vi "TLB Native Dynamic Events ver 0.26d.vi"() -> ()   [LabVIEW 2018] (continued)
      tunnel: [_ _ _ _ _ _ _ _ _ _ _ _ _ _ _ _ _ _ _ _ _ _ _ _ _ _ _ _ _ _ _ _ _ _ _ w3525 w3555 _ _ _ _ _ _ _ _ _ _ _ _ _ _ _ _ _ _ _ _] -> w221
      tunnel: w219 -> [w2959 w2972 w2984 w2999 w3018 w3033 w3048 w3062 w3076 w3092 w3107 w3121 w3132 w3149 w3167 w3185 w3201 w3220 w3232 w3262 w3275 w3288 w3303 w3314 w3333 w3353 w3388 w3419 w3432 w3445 w3456 w3468 w3484 w3500 w3512 w3524 w3559 w3570 w3582 w3603 w3614 w3625 w3638 w3651 w3664 w3677 w3690 w3705 w3721 w3734 w3750 w3766 w3782 w3799 w3812 w3832 w3852]
      tunnel: [w2959 w2972 w2984 w2999 w3018 w3033 w3048 w3062 w3076 w3092 w3107 w3121 w3132 w3149 w3167 w3185 w3201 w3220 w3232 w3262 w3275 w3288 w3303 w3314 w3333 w3353 w3388 w3419 w3432 w3445 w3456 w3468 w3484 w3500 w3512 w3524 w3559 w3570 w3582 w3603 w3614 w3625 w3638 w3651 w3664 w3677 w3690 w3705 w3721 w3734 w3750 w3766 w3782 w3799 w3812 w3832 w3852] -> w218
      tunnel: w214 -> [w2958 w2971 w2983 w2998 w3017 w3032 w3047 w3061 w3075 w3091 w3106 w3120 w3131 w3148 w3166 w3182 w3200 w3219 w3231 w3261 w3274 w3287 w3302 w3313 w3328 w3346 w3381 w3418 w3431 w3444 w3455 w3467 w3483 w3499 w3511 w3523 w3553 w3569 w3581 w3602 w3613 w3624 w3637 w3650 w3663 w3676 w3689 w3704 w3720 w3733 w3749 w3765 w3781 w3798 w3811 w3831 w3846]
      tunnel: [w2958 w2971 w2983 w2998 w3017 w3032 w3047 w3061 w3075 w3091 w3106 w3120 w3131 w3148 w3166 w3182 w3200 w3219 w3231 w3261 w3274 w3287 w3302 w3313 w3327 w3346 w3381 w3418 w3431 w3444 w3455 w3467 w3483 w3499 w3511 w3523 w3546 w3569 w3581 w3601 w3613 w3624 w3637 w3650 w3663 w3676 w3689 w3704 w3720 w3733 w3749 w3765 w3781 w3798 w3811 w3831 w3845] -> w213
      frame "Exit" {
        # ">>State Logic  >>"
        # ">>> Time cluster >>>"
        # ">>> Yaw >>>"
        # ">>> Stepper position >>>"
        # ">>> Encoders >>>"
        # ">>> Object detection >>>"
        # ">>> Ultrasonic Sensors Detect >>>"
        n70 = call "Imaq Dispose"("All Images? (No)"=TRUE) -> ()  [unwired: 5 in, 1 out]
      }
      frame "----Movement States----" {
        # ">>State Logic  >>"
        # ">>> Time cluster >>>"
        # ">>> Yaw >>>"
        # ">>> Stepper position >>>"
        # ">>> Encoders >>>"
        # ">>> Object detection >>>"
        # ">>> Ultrasonic Sensors Detect >>>"
      }
      frame "FORWARD" {
        # ">>State Logic  >>"
        # ">>> Time cluster >>>"
        # ">>> Yaw >>>"
        # ">>> Stepper position >>>"
        # ">>> Encoders >>>"
        # ">>> Object detection >>>"
        # ">>> Ultrasonic Sensors Detect >>>"
        n71 = Unbundle By Name(w2991) -> ("Yaw"=w2987:dbl)
        n72 = call "MOTOR CONTROL WITH PID AE.vi"("Yaw"=w2987, "Speed"=50.0, "Direction"=MOTOR_CONTROL_WITH_PID_AE_DIRECTION_TYPE_DEF."y-axis movement", "AE Mode"=MOTOR_CONTROL_WITH_PID_AE_DATA_MODE_TYPE_DEF."Write to AE") -> ()  [unwired: 1 out]
      }
      frame "FORWARD - IR ASSIST" {
        # "Algorithm sensitivity"
        # "Distance to maintain from wall"
        # ">>State Logic  >>"
        # ">>> Time cluster >>>"
        # ">>> Yaw >>>"
        # ">>> Stepper position >>>"
        # ">>> Encoders >>>"
        # ">>> Object detection >>>"
        # ">>> Ultrasonic Sensors Detect >>>"
        n73 = Unbundle By Name(w3006) -> ("Left IR Sensor"=w3005:dbl)
        n74 = Subtract(x=w3005, y=10.0) -> (x-y=w3003:dbl)
        n75 = Multiply(x=w3003, y=0.2) -> (x*y=w3001:dbl)
        n76 = call "MOTOR CONTROL WITH PID AE.vi"("Yaw"=w3001, "Speed"=35.0, "Direction"=MOTOR_CONTROL_WITH_PID_AE_DIRECTION_TYPE_DEF."y-axis movement", "AE Mode"=MOTOR_CONTROL_WITH_PID_AE_DATA_MODE_TYPE_DEF."Write to AE") -> ()  [unwired: 1 out]
      }
      frame "LEFT" {
        # ">>State Logic  >>"
        # ">>> Time cluster >>>"
        # ">>> Yaw >>>"
        # ">>> Stepper position >>>"
        # ">>> Encoders >>>"
        # ">>> Object detection >>>"
        # ">>> Ultrasonic Sensors Detect >>>"
        n77 = Unbundle By Name(w3025) -> ("Yaw"=w3022:dbl)
        n78 = call "MOTOR CONTROL WITH PID AE.vi"("Yaw"=w3022, "Speed"=-20.0, "Direction"=MOTOR_CONTROL_WITH_PID_AE_DIRECTION_TYPE_DEF."x-axis movement", "AE Mode"=MOTOR_CONTROL_WITH_PID_AE_DATA_MODE_TYPE_DEF."Write to AE") -> ()  [unwired: 1 out]
      }
      frame "RIGHT" {
        # ">>> Time cluster >>>"
        # ">>> Yaw >>>"
        # ">>> Stepper position >>>"
        # ">>> Encoders >>>"
        # ">>> Object detection >>>"
        # ">>> Ultrasonic Sensors Detect >>>"
        n79 = Unbundle By Name(w3040) -> ("Yaw"=w3036:dbl)
        n80 = call "MOTOR CONTROL WITH PID AE.vi"("Yaw"=w3036, "Speed"=20.0, "Direction"=MOTOR_CONTROL_WITH_PID_AE_DIRECTION_TYPE_DEF."x-axis movement", "AE Mode"=MOTOR_CONTROL_WITH_PID_AE_DATA_MODE_TYPE_DEF."Write to AE") -> ()  [unwired: 1 out]
      }
      frame "R-ACW" {
        # ">>> IR Sensors >>>"
        # ">>> Time cluster >>>"
        # ">>> Yaw >>>"
        # ">>> Stepper position >>>"
        # ">>> Encoders >>>"
        # ">>> Object detection >>>"
        # ">>> Ultrasonic Sensors Detect >>>"
        n81 = call "MOTOR CONTROL WITH PID AE.vi"("Speed"=10.0, "Direction"=MOTOR_CONTROL_WITH_PID_AE_DIRECTION_TYPE_DEF."rotation", "AE Mode"=MOTOR_CONTROL_WITH_PID_AE_DATA_MODE_TYPE_DEF."Write to AE") -> ()  [unwired: 1 in, 1 out]
      }
      frame "R-CW" {
        (unwired) -0.2 ("Speed")
        # ">>> Time cluster >>>"
        # ">>> Yaw >>>"
        # ">>> Stepper position >>>"
        # ">>> Encoders >>>"
        # ">>> Object detection >>>"
        # ">>> Ultrasonic Sensors Detect >>>"
        n82 = call "MOTOR CONTROL WITH PID AE.vi"("Speed"=-10.0, "Direction"=MOTOR_CONTROL_WITH_PID_AE_DIRECTION_TYPE_DEF."rotation", "AE Mode"=MOTOR_CONTROL_WITH_PID_AE_DATA_MODE_TYPE_DEF."Write to AE") -> ()  [unwired: 1 in, 1 out]
      }
      frame "X AXIS - SLOW" {
        # ">>> Line Sensor Cluster>>>"
        # ">>> IR Sensors >>>"
        # ">>> Time cluster >>>"
        # ">>> Yaw >>>"
        # ">>> Stepper position >>>"
        # ">>> Encoders >>>"
        # ">>> Object detection >>>"
        # ">>> Ultrasonic Sensors Detect >>>"
        n83 = Unbundle By Name(w3079) -> ("xSpeed"=w3078:dbl)
        n84 = Unbundle By Name(w3084) -> ("Yaw"=w3081:dbl)
        n85 = call "MOTOR CONTROL WITH PID AE.vi"("Yaw"=w3081, "Speed"=w3078, "Direction"=MOTOR_CONTROL_WITH_PID_AE_DIRECTION_TYPE_DEF."x-axis movement", "AE Mode"=MOTOR_CONTROL_WITH_PID_AE_DATA_MODE_TYPE_DEF."Write to AE") -> ()  [unwired: 1 out]
      }
      frame "REVERSE" {
        # ">>> Time cluster >>>"
        # ">>> Yaw >>>"
        # ">>> Stepper position >>>"
        # ">>> Encoders >>>"
        # ">>> Object detection >>>"
        # ">>> Ultrasonic Sensors Detect >>>"
        n86 = Unbundle By Name(w3099) -> ("Yaw"=w3095:dbl)
        n87 = call "MOTOR CONTROL WITH PID AE.vi"("Yaw"=w3095, "Speed"=-50.0, "Direction"=MOTOR_CONTROL_WITH_PID_AE_DIRECTION_TYPE_DEF."y-axis movement", "AE Mode"=MOTOR_CONTROL_WITH_PID_AE_DATA_MODE_TYPE_DEF."Write to AE") -> ()  [unwired: 1 out]
      }
      frame "STOP" {
        n88 = Wait (ms)(milliseconds to wait=u32 100) -> ()  [unwired: 1 out]
        n89 = call "MOTOR CONTROL WITH PID AE.vi"("Direction"=MOTOR_CONTROL_WITH_PID_AE_DIRECTION_TYPE_DEF."stop", "AE Mode"=MOTOR_CONTROL_WITH_PID_AE_DATA_MODE_TYPE_DEF."Write to AE") -> ()  [unwired: 2 in, 1 out]
      }
      frame "----SENSOR READING---- " {
      }
      frame "READ ENCODERS" {
        # ">>> Time cluster >>>"
        # ">>> Yaw >>>"
        # ">>> Stepper position >>>"
        # ">>> Object detection >>>"
        # ">>> Current encoder distance >>>"
        # ">>> Ultrasonic Sensors Detect >>>"
        n90 = call "MOTOR CONTROL WITH PID AE.vi"("AE Mode"=MOTOR_CONTROL_WITH_PID_AE_DATA_MODE_TYPE_DEF."Read from AE") -> ("Speed & distance"=w3138:T15)  [unwired: 3 in]
        n91 = Unbundle By Name(w3138) -> ("xDistance"=w3137:dbl, "yDistance"=w3136:dbl, "wDistance"=w3135:dbl)
        n92 = Bundle By Name(cluster=w3145, "xDistance"=w3137, "yDistance"=w3136, "wDistance"=w3135) -> (w3144:T8)
      }
      frame "READ ULTRASONIC" {
        (unwired) navX_type_def."Read Values" ("Mode")
        (unwired) MOTOR_CONTROL_NO_PID_Type_Def."Latch" ("Direction")
        # ">>> Line Sensor Cluster>>>"
        # ">>> IR Sensors >>>"
        # ">>State Logic  >>"
        # ">>> Time cluster >>>"
        # ">>> Ultrasonic Sensors Detect >>>"
        # ">>> Object detection >>>"
        # ">>> Encoders >>>"
        # ">>> Stepper position >>>"
        # ">>> Yaw >>>"
        n93 = call "Arduino Interfacing VI.vi"("AE Mode"=Arduino_Interfacing."Read From Arduino") -> ("Arduino Data"=w3158:T17)  [unwired: 3 in, 1 out]
        n94 = Unbundle By Name(w3158) -> ("PING A"=w3157:u8, "PING B"=w3156:u8, "PING C"=w3155:u8, "PING D"=w3154:u8)
        n95 = Bundle By Name(cluster=w3164, "PING_A"=w3157, "PING_B"=w3156, "PING_C"=w3155, "PING_D"=w3154) -> (w3165:T9)
      }
      frame "READ NAVX" {
        # ">> Item Selection Bias >>"
        # ">>State Logic  >>"
        # ">>> Line Sensor Cluster>>>"
        # ">>> IR Sensors >>>"
        # ">>> Time cluster >>>"
        # ">>> Yaw >>>"
        # ">>> Ultrasonic Sensors Detect >>>"
        # ">>> Object detection >>>"
        # ">>> Encoders >>>"
        # ">>> Stepper position >>>"
        n96 = call "navX reading VI.vi"("Mode"=navX_type_def."Read Values") -> ("NavX Readings"=w3171:T16)  [unwired: 2 in, 3 out]
        n97 = Unbundle By Name(w3171) -> ("Heading"=w3170:dbl)
        n98 = Unbundle By Name(w3171) -> ("Yaw"=w3174:dbl)
        n99 = Bundle By Name(cluster=w3176, "Yaw"=w3174, "Compass"=w3170) -> (w3175:T6)
      }
      frame "READ IR" {
        w3184 = T41 [enum."B/AI2"] items=["Not Connected", "AudioIn/Left", "AudioIn/Right", "C/AI0", "C/AI1", "A/AI0", "A/AI1", "A/AI2", "A/AI3", "A/AI4", "A/AI5", "A/AI6", "A/AI7", "B/AI0", "B/AI1", "B/AI2", "B/AI3", "B/AI4", "B/AI5", "B/AI6", "B/AI7", "AI/AI0", "AI/AI1", "AI/AI2", "AI/AI3", "A/AI0 (DIFF)", "A/AI1 (DIFF)", "A/AI2 (DIFF)", "A/AI3 (DIFF)", "B/AI0 (DIFF)", "B/AI1 (DIFF)", "B/AI2 (DIFF)", "B/AI3 (DIFF)"] ("AI Channel")
        w3188 = T41 [enum."B/AI1"] items=["Not Connected", "AudioIn/Left", "AudioIn/Right", "C/AI0", "C/AI1", "A/AI0", "A/AI1", "A/AI2", "A/AI3", "A/AI4", "A/AI5", "A/AI6", "A/AI7", "B/AI0", "B/AI1", "B/AI2", "B/AI3", "B/AI4", "B/AI5", "B/AI6", "B/AI7", "AI/AI0", "AI/AI1", "AI/AI2", "AI/AI3", "A/AI0 (DIFF)", "A/AI1 (DIFF)", "A/AI2 (DIFF)", "A/AI3 (DIFF)", "B/AI0 (DIFF)", "B/AI1 (DIFF)", "B/AI2 (DIFF)", "B/AI3 (DIFF)"] ("AI Channel")
        w3193 = T41 [enum."B/AI0"] items=["Not Connected", "AudioIn/Left", "AudioIn/Right", "C/AI0", "C/AI1", "A/AI0", "A/AI1", "A/AI2", "A/AI3", "A/AI4", "A/AI5", "A/AI6", "A/AI7", "B/AI0", "B/AI1", "B/AI2", "B/AI3", "B/AI4", "B/AI5", "B/AI6", "B/AI7", "AI/AI0", "AI/AI1", "AI/AI2", "AI/AI3", "A/AI0 (DIFF)", "A/AI1 (DIFF)", "A/AI2 (DIFF)", "A/AI3 (DIFF)", "B/AI0 (DIFF)", "B/AI1 (DIFF)", "B/AI2 (DIFF)", "B/AI3 (DIFF)"] ("AI Channel")
        # ">>> Line Sensor Cluster>>>"
        # ">>> IR Sensors >>>"
        # ">>State Logic  >>"
        # ">>> Time cluster >>>"
        # ">>> Ultrasonic Sensors Detect >>>"
        # ">>> Object detection >>>"
        # ">>> Encoders >>>"
        # ">>> Stepper position >>>"
        # ">>> Yaw >>>"
        n100 = call <vilib>:"Sharp IR.vi"("AI Channel"=w3193) -> ("Sharp IR Distance"=w3189:dbl)  [unwired: 8 in, 2 out]
        n101 = call <vilib>:"Sharp IR.vi"("AI Channel"=w3188) -> ("Sharp IR Distance"=w3187:dbl)  [unwired: 8 in, 2 out]
        n102 = call <vilib>:"Sharp IR.vi"("AI Channel"=w3184) -> ("Sharp IR Distance"=w3183:dbl)  [unwired: 8 in, 2 out]
        n103 = Bundle By Name(cluster=w3191, "Left IR Sensor"=w3189, "Arm IR Sensor"=w3187, "Bottom IR Sensor"=w3183) -> (w3190:T5)
      }
      frame "READ LINE SENSOR" {
        # ">>> IR Sensors >>>"
        # ">>> Line Sensor Cluster>>>"
        # ">>State Logic  >>"
        # ">>> Time cluster >>>"
        # ">>> Object detection >>>"
        # ">>> Yaw >>>"
        # ">>> Ultrasonic Sensors Detect >>>"
        # ">>> Encoders >>>"
        # ">>> Stepper position >>>"
        n104 = call "Line Sensor AE.vi"("AE State"=Line_Sensor_AE_Type_Def."READ FROM LINE SENSORS") -> ("Line Detected?"=w3207:bool, "Line Sensor Raw Values"=w3206:T43)
        n105 = Unbundle By Name(w3206) -> ("S1"=w3205:dbl, "S2"=w3204:dbl, "S3"=w3203:dbl, "S4"=w3202:dbl)
        n106 = Bundle By Name(cluster=w3210, "Line Detected?"=w3207, "S1"=w3205, "S2"=w3204, "S3"=w3203, "S4"=w3202) -> (w3209:T4)
      }
      frame "----SYSTEM MODES----" {
        (unwired) I2C_MASTER_Type_Def."Last State" ("Arduino Mode")
        # ">>> Object detection >>>"
        # ">>> Yaw >>>"
        # ">>> Ultrasonic Sensors Detect >>>"
        # ">>> Encoders >>>"
        # ">>> Stepper position >>>"
      }
      frame "INIT" {
        w3254 = u8 0
        w3255 = 0.0
        # ">>> IR Sensors >>>"
        # ">>> IR Sensors >>>"
        # ">>> Line Sensor Cluster>>>"
        # ">>> Time cluster >>>"
        # ">>> Object detection >>>"
        # ">>> Yaw >>>"
        # ">>> Ultrasonic Sensors Detect >>>"
        # ">>> Encoders >>>"
        # ">>> Stepper position >>>"
        # ">>State Logic  >>"
        n107 = call "Arduino Interfacing VI.vi"("AE Mode"=Arduino_Interfacing."Initialize") -> ()  [unwired: 3 in, 2 out]
        n108 = call "FGV Stop.vi"("Init/Read/Write State"=States_for_Action_Engine."Initialize") -> ()  [unwired: 2 in, 2 out]
        n109 = call "Elasped Timer.vi"("Action"=Elapsed_timer_control."Initialize") -> ()  [unwired: 7 in, 4 out]
        n110 = call "MOTOR CONTROL WITH PID AE.vi"("AE Mode"=MOTOR_CONTROL_WITH_PID_AE_DATA_MODE_TYPE_DEF."Init AE") -> ()  [unwired: 3 in, 1 out]
        n111 = call "IMAQ Reference AE.vi"("IMAQ AE States"=IMAQ_Reference_AE."Initialize AE") -> ()  [unwired: 1 in, 2 out]
        n112 = call "Line Sensor AE.vi"("AE State"=Line_Sensor_AE_Type_Def."INIT AE") -> ()  [unwired: 2 out]
        n113 = Bundle By Name(cluster=w3248, "Recognized Object"=FALSE, "Object X coordinate"=0.0, "Object Y coordinate"=0.0) -> (w3247:T11)
        n114 = Bundle By Name(cluster=w3253, "y Stepper Position"=u8 0, "z Stepper Position"=u8 0) -> (w3252:T7)
        n115 = Bundle By Name(cluster=w3257, "xDistance"=w3255, "yDistance"=w3255, "wDistance"=w3255) -> (w3256:T8)
        n116 = Bundle By Name(cluster=w3259, "PING_A"=w3254, "PING_B"=w3254, "PING_C"=w3254, "PING_D"=w3254) -> (w3260:T9)
        n117 = Bundle By Name(cluster=w3243, "Yaw"=0.0) -> (w3242:T6)
        n118 = call "Task 9 basic VI.vi"("AE State"=Task_9_Sates."Initialize") -> ()  [unwired: 1 in, 3 out]
      }
      frame "ARDUINO - ULTRASONIC" {
        # ">>> Time cluster >>>"
        # ">>> Line Sensor Cluster>>>"
        # ">>> Object detection >>>"
        # ">>> Yaw >>>"
        # ">>> Ultrasonic Sensors Detect >>>"
        # ">>> Encoders >>>"
        # ">>> Stepper position >>>"
        # ">>State Logic  >>"
        n119 = call "Arduino Interfacing VI.vi"("Data to Write"=I2C_MASTER_WRITE_NEW_Type_Def."Ultrasonic sensors", "AE Mode"=Arduino_Interfacing."Write to Arduino") -> ()  [unwired: 2 in, 2 out]
      }
      frame "NAVX CALIBRATE" {
        # ">>> Object detection >>>"
        # ">>> Yaw >>>"
        # ">>> Ultrasonic Sensors Detect >>>"
        # ">>> Encoders >>>"
        # ">>> Stepper position >>>"
        # ">>State Logic  >>"
        # "Adds a 15 second delay to the startup process \nfor the NavX to calibrate"
        n120 = Wait (ms)(milliseconds to wait=u32 1000) -> ()  [unwired: 1 out]
      }
      frame "NO ACTION", Default {
        (unwired) u8 0 ("y Stepper value")
        (unwired) TRUE ("Latch")
        (unwired) navX_type_def."Read Values" ("Mode")
        (unwired) MOTOR_CONTROL_NO_PID_Type_Def."Latch" ("Direction")
        # ">>> Object detection >>>"
        # ">>> Yaw >>>"
        # ">>> Ultrasonic Sensors Detect >>>"
        # ">>> Encoders >>>"
        # ">>> Stepper position >>>"
        # ">>State Logic  >>"
        n121 = case shown="4" w3296 {
          tunnel: [0 100] -> w3298
          frame 1, Default {
          }
          frame 4 {
          }
        }
      }
      frame "----RESET CASES----" {
        (unwired) I2C_MASTER_Type_Def."Last State" ("Arduino Mode")
        # ">>> Object detection >>>"
        # ">>> Yaw >>>"
        # ">>> Ultrasonic Sensors Detect >>>"
        # ">>> Encoders >>>"
        # ">>> Stepper position >>>"
        # ">>State Logic  >>"
      }
      frame "RESET ENCODERS" {
        # ">>> Object detection >>>"
        # ">>> Yaw >>>"
        # ">>> Ultrasonic Sensors Detect >>>"
        # ">>> Encoders >>>"
        # ">>> Stepper position >>>"
        # ">>State Logic  >>"
        n122 = call "MOTOR CONTROL WITH PID AE.vi"("Direction"=MOTOR_CONTROL_WITH_PID_AE_DIRECTION_TYPE_DEF."reset encoders", "AE Mode"=MOTOR_CONTROL_WITH_PID_AE_DATA_MODE_TYPE_DEF."Write to AE") -> ()  [unwired: 2 in, 1 out]
      }
      frame "RESET FLAGS" {
        w3326 = FALSE ("Line Detected?")
        # ">>> Line Sensor Cluster>>>"
        # ">>> IR Sensors >>>"
        # ">>> Time cluster >>>"
        # ">>> Object detection >>>"
        # ">>> Yaw >>>"
        # ">>> Ultrasonic Sensors Detect >>>"
        # ">>> Encoders >>>"
        # ">>> Stepper position >>>"
        # ">>> Line Sensor Cluster>>>"
        # ">>> IR Sensors >>>"
        # ">>> Time cluster >>>"
        # ">>> Object detection >>>"
        # ">>> Yaw >>>"
        # ">>> Ultrasonic Sensors Detect >>>"
        # ">>> Encoders >>>"
        # ">>> Stepper position >>>"
        # "Resets BOOLEAN FLAGS only"
        n123 = Wait (ms)(milliseconds to wait=u32 20) -> ()  [unwired: 1 out]
        n124 = Bundle By Name(cluster=w3342, "Recognized Object"=FALSE) -> (w3341:T11)
        n125 = Bundle By Name(cluster=w3332, "Line Detected?"=FALSE) -> (w3331:T4)
        n126 = Bundle By Name(cluster=w3336, "Time up flag"=FALSE) -> (w3335:T3)
        n127 = Bundle By Name(cluster=w3328, "Red"=w3326, "Black"=w3326, "Blue"=w3326, "Yellow"=w3326, "Green"=w3326, "Unknown"=w3326, "Image processing done"=w3326) -> (w3327:T1)
      }
      frame "RESET SENSOR VALUES" {
        w3347 = 0.0 ("S4")
        w3348 = 0.0 ("S4")
        # "Resets SENSOR VALUES only"
        # ">>> Line Sensor Cluster>>>"
        # ">>> IR Sensors >>>"
        # ">>> Time cluster >>>"
        # ">>> Object detection >>>"
        # ">>> Yaw >>>"
        # ">>> Ultrasonic Sensors Detect >>>"
        # ">>> Encoders >>>"
        # ">>> Stepper position >>>"
        # ">>> Line Sensor Cluster>>>"
        # ">>> IR Sensors >>>"
        # ">>> Time cluster >>>"
        # ">>> Object detection >>>"
        # ">>> Yaw >>>"
        # ">>> Ultrasonic Sensors Detect >>>"
        # ">>> Encoders >>>"
        # ">>> Stepper position >>>"
        # "Resets any software variables\nand/or non-critical states"
        n128 = Wait (ms)(milliseconds to wait=u32 20) -> ()  [unwired: 1 out]
        n129 = Bundle By Name(cluster=w3356, "SET TIME TO CHECK"=0.0) -> (w3355:T3)
        n130 = Bundle By Name(cluster=w3372, "Object X coordinate"=0.0, "Object Y coordinate"=0.0) -> (w3371:T11)
        n131 = Bundle By Name(cluster=w3363, "y Stepper Position"=u8 0, "z Stepper Position"=u8 0) -> (w3362:T7)
        n132 = Bundle By Name(cluster=w3350, "Left IR Sensor"=w3347, "Arm IR Sensor"=w3347) -> (w3349:T5)
        n133 = Bundle By Name(cluster=w3368, "xDistance"=0.0, "yDistance"=0.0, "wDistance"=0.0) -> (w3367:T8)
        n134 = Bundle By Name(cluster=w3379, "PING_A"=u8 0, "PING_B"=u8 0, "PING_C"=u8 0, "PING_D"=u8 0) -> (w3378:T9)
        n135 = Bundle By Name(cluster=w3359, "Yaw"=0.0) -> (w3358:T6)
        n136 = Bundle By Name(cluster=w3352, "S1"=w3348, "S2"=w3348, "S3"=w3348, "S4"=w3348) -> (w3351:T4)
      }
      frame "RESET ALL SENSORS" {
        w3382 = 0.0 ("SET TIME TO CHECK")
        # ">>> Line Sensor Cluster>>>"
        # ">>> IR Sensors >>>"
        # ">>> Time cluster >>>"
        # ">>> Object detection >>>"
        # ">>> Yaw >>>"
        # ">>> Ultrasonic Sensors Detect >>>"
        # ">>> Encoders >>>"
        # ">>> Stepper position >>>"
        # ">>> Line Sensor Cluster>>>"
        # ">>> IR Sensors >>>"
        # ">>> Time cluster >>>"
        # ">>> Object detection >>>"
        # ">>> Yaw >>>"
        # ">>> Ultrasonic Sensors Detect >>>"
        # ">>> Encoders >>>"
        # ">>> Stepper position >>>"
        # "Resets ALL SENSOR PARAMTERS"
        n137 = Wait (ms)(milliseconds to wait=u32 20) -> ()  [unwired: 1 out]
        n138 = Bundle By Name(cluster=w3392, "Time up flag"=FALSE, "SET TIME TO CHECK"=0.0) -> (w3391:T3)
        n139 = Bundle By Name(cluster=w3409, "Recognized Object"=FALSE, "Object X coordinate"=0.0, "Object Y coordinate"=0.0) -> (w3408:T11)
        n140 = Bundle By Name(cluster=w3399, "y Stepper Position"=u8 0, "z Stepper Position"=u8 0) -> (w3398:T7)
        n141 = Bundle By Name(cluster=w3387, "Line Detected?"=FALSE) -> (w3386:T4)
        n142 = Bundle By Name(cluster=w3384, "Left IR Sensor"=w3382, "Arm IR Sensor"=w3382) -> (w3383:T5)
        n143 = Bundle By Name(cluster=w3404, "xDistance"=0.0, "yDistance"=0.0, "wDistance"=0.0) -> (w3403:T8)
        n144 = Bundle By Name(cluster=w3416, "PING_A"=u8 0, "PING_B"=u8 0, "PING_C"=u8 0, "PING_D"=u8 0) -> (w3415:T9)
        n145 = Bundle By Name(cluster=w3395, "Yaw"=0.0) -> (w3394:T6)
      }
      frame "RESET YAW" {
        n146 = Wait (ms)(milliseconds to wait=u32 100) -> ()  [unwired: 1 out]
        n147 = call "navX reading VI.vi"("Mode"=navX_type_def."Zero Yaw") -> ()  [unwired: 2 in, 4 out]
      }
      frame "RESET ARM" {
        n148 = call "Arduino Interfacing VI.vi"("Data to Write"=I2C_MASTER_WRITE_NEW_Type_Def."Soft Reset", "AE Mode"=Arduino_Interfacing."Write to Arduino") -> ()  [unwired: 2 in, 2 out]
      }
      frame "--------CAM STATES-------" {
      }
      frame "OPEN IMAQ REF" {
        # ">>> Line Sensor Cluster>>>"
        # ">>State Logic  >>"
        # ">>> Time cluster >>>"
        # ">>> Object detection >>>"
        # ">>> Yaw >>>"
        # ">>> Ultrasonic Sensors Detect >>>"
        # ">>> Encoders >>>"
        # ">>> Stepper position >>>"
        # ">>> IR Sensors >>>"
        n149 = call "IMAQ Reference AE.vi"("IMAQ AE States"=IMAQ_Reference_AE."Initialize AE") -> ()  [unwired: 1 in, 2 out]
      }
      frame "OPEN LOG CAM" {
        n150 = call "Webcam AE.vi"("Session In"=T39 "cam0", "Camera states"=Webcam_AE."Initialize Camera") -> ("error out"=w3473:errorcluster, "Session Out"=w3472:T39)  [unwired: 1 in, 1 out]
        n151 = call "Webcam AE.vi"("error in (no error)"=w3473, "Session In"=w3472, "Camera states"=Webcam_AE."Open Camera") -> ()  [unwired: 3 out]
      }
      frame "OPEN LIFE CAM" {
        n152 = call "Webcam AE.vi"("Session In"=T39 "cam1", "Camera states"=Webcam_AE."Initialize Camera") -> ("error out"=w3489:errorcluster, "Session Out"=w3488:T39)  [unwired: 1 in, 1 out]
        n153 = call "Webcam AE.vi"("error in (no error)"=w3489, "Session In"=w3488, "Camera states"=Webcam_AE."Open Camera") -> ()  [unwired: 3 out]
      }
      frame "CAM ACQ" {
        # ">>State Logic  >>"
        # ">>> Time cluster >>>"
        # ">>> Yaw >>>"
        # ">>> Stepper position >>>"
        # ">>> Encoders >>>"
        # ">>> Object detection >>>"
        # ">>> Ultrasonic Sensors Detect >>>"
        n154 = call "Webcam AE.vi"("Camera states"=Webcam_AE."Continuous Acquisition") -> ()  [unwired: 2 in, 3 out]
      }
      frame "CAM CLOSE" {
        # ">>> Box Colour Detection >>>"
        # ">>> Line Sensor Cluster>>>"
        # ">>> IR Sensors >>>"
        # ">>State Logic  >>"
        # ">>> Time cluster >>>"
        # ">>> Yaw >>>"
        # ">>> Stepper position >>>"
        # ">>> Encoders >>>"
        # ">>> Object detection >>>"
        # ">>> Ultrasonic Sensors Detect >>>"
        n155 = call "Webcam AE.vi"("Camera states"=Webcam_AE."Close Camera") -> ()  [unwired: 2 in, 3 out]
      }
      frame "PROCESS IMAGE" {
        # ">>> Line Sensor Cluster>>>"
        # ">>> IR Sensors >>>"
        # ">> Item Selection Bias >>"
        # ">> Item Selection Bias >>"
        # ">>State Logic  >>"
        # ">>> Time cluster >>>"
        # ">>> Yaw >>>"
        # ">>> Stepper position >>>"
        # ">>> Encoders >>>"
        # ">>> Object detection >>>"
        # ">>> Ultrasonic Sensors Detect >>>"
        n156 = call "Webcam AE.vi"("Camera states"=Webcam_AE."Retrieve Image") -> ("error out"=w3537:errorcluster, "Image Out"=w3538:T45)  [unwired: 2 in, 1 out]
        n157 = call "IMAQ Reference AE.vi"("IMAQ AE States"=IMAQ_Reference_AE."Get IMAQ Reference") -> ("Image Out"=w3527:T45)  [unwired: 1 in, 1 out]
        n158 = call "Object Detection SubVI.vi"("Error In"=w3537, "Mode"=w3524, "Image Dest"=w3527, "Image in"=w3538) -> ("Error out"=w3525:errorcluster, "Object Center Coordinates"=w3534:cluster{"x":sgl, "y":sgl}, "Object detection cluster"=w3530:T46)  [unwired: 1 out]
        n159 = Unbundle By Name(w3530) -> ("Object detected?"=w3531:bool)
        n160 = Unbundle By Name(w3534) -> ("x"=w3533:sgl, "y"=w3532:sgl)
        n161 = Bundle By Name(cluster=w3536, "Recognized Object"=w3531, "Object X coordinate"=w3533, "Object Y coordinate"=w3532) -> (w3535:T11)
      }
      frame "COLOUR PROCESSING" {
        # ">>> Box Colour Detection >>>"
        # ">>> Box Colour Detection >>>"
        # ">>> Line Sensor Cluster>>>"
        # ">>> IR Sensors >>>"
        # ">> Item Selection Bias >>"
        # ">> Item Selection Bias >>"
        # ">>State Logic  >>"
        # ">>> Time cluster >>>"
        # ">>> Yaw >>>"
        # ">>> Stepper position >>>"
        # ">>> Encoders >>>"
        # ">>> Object detection >>>"
        # ">>> Ultrasonic Sensors Detect >>>"
        n162 = call "Webcam AE.vi"("Camera states"=Webcam_AE."Retrieve Image") -> ("error out"=w3556:errorcluster, "Image Out"=w3557:T45)  [unwired: 2 in, 1 out]
        n163 = call "Box Colour Detection SubVI.vi"("Image In"=w3557, "Error In"=w3556) -> ("Colour output boolean cluster"=w3554:T47, "Error out"=w3555:errorcluster)  [unwired: 1 out]
        n164 = Unbundle By Name(w3554) -> ("Red"=w3552:bool, "Black"=w3551:bool, "Blue"=w3550:bool, "Yellow"=w3549:bool, "Green"=w3548:bool, "No recognizable coolour"=w3547:bool)
        n165 = Bundle By Name(cluster=w3553, "Red"=w3552, "Black"=w3551, "Blue"=w3550, "Yellow"=w3549, "Green"=w3548, "Unknown"=w3547) -> (w3546:T1)
      }
      frame "DISPOSE CAM BUFFERS" {
        # ">> Item Selection Bias >>"
        # ">>> Line Sensor Cluster>>>"
        # ">>> IR Sensors >>>"
        # ">>State Logic  >>"
        # ">>> Time cluster >>>"
        # ">>> Yaw >>>"
        # ">>> Stepper position >>>"
        # ">>> Encoders >>>"
        # ">>> Object detection >>>"
        # ">>> Ultrasonic Sensors Detect >>>"
        n166 = call "Webcam AE.vi"("Camera states"=Webcam_AE."Dispose Camera Image Buffer") -> ()  [unwired: 2 in, 3 out]
      }
      frame "DISPOSE PROC BUFFERS" {
        # ">>> Box Colour Detection >>>"
        # ">>> Line Sensor Cluster>>>"
        # ">>State Logic  >>"
        # ">>> IR Sensors >>>"
        # ">>> Time cluster >>>"
        # ">>> Object detection >>>"
        # ">>> Yaw >>>"
        # ">>> Ultrasonic Sensors Detect >>>"
        # ">>> Encoders >>>"
        # ">>> Stepper position >>>"
        n167 = call "IMAQ Reference AE.vi"("IMAQ AE States"=IMAQ_Reference_AE."Dispose Processing Buffer") -> ()  [unwired: 1 in, 2 out]
      }
      frame "BOX COLOUR" {
        # ">>> Box Colour Detection >>>"
        # ">>> Line Sensor Cluster>>>"
        # ">>State Logic  >>"
        # ">>> IR Sensors >>>"
        # ">>> Time cluster >>>"
        # ">>> Object detection >>>"
        # ">>> Yaw >>>"
        # ">>> Ultrasonic Sensors Detect >>>"
        # ">>> Encoders >>>"
        # ">>> Stepper position >>>"
        n168 = call "Box Colour Detection Sequence.vi"() -> ("Colour scan time out?"=w3593:bool, "Colour output boolean cluster"=w3600:T47)  [unwired: 9 in, 1 out]
        n169 = Unbundle By Name(w3600) -> ("Red"=w3599:bool, "Black"=w3598:bool, "Blue"=w3597:bool, "Yellow"=w3596:bool, "Green"=w3595:bool, "No recognizable coolour"=w3594:bool)
        n170 = Bundle By Name(cluster=w3602, "Red"=w3599, "Black"=w3598, "Blue"=w3597, "Yellow"=w3596, "Green"=w3595, "Unknown"=w3594, "Image processing done"=w3593) -> (w3601:T1)
      }
      frame "-----ARM ACTIONS-----" {
      }
      frame "CLOSE CLAW" {
        n171 = call "Arduino Interfacing VI.vi"("Data to Write"=I2C_MASTER_WRITE_NEW_Type_Def."Close Claw", "AE Mode"=Arduino_Interfacing."Write to Arduino") -> ()  [unwired: 2 in, 2 out]
      }
      frame "OPEN CLAW" {
        n172 = call "Arduino Interfacing VI.vi"("Data to Write"=I2C_MASTER_WRITE_NEW_Type_Def."Open Claw", "AE Mode"=Arduino_Interfacing."Write to Arduino") -> ()  [unwired: 2 in, 2 out]
      }
      frame "Z STEPPER CAM HEIGHT" {
        n173 = call "Arduino Interfacing VI.vi"("Data to Write"=I2C_MASTER_WRITE_NEW_Type_Def."zStepper 6k", "AE Mode"=Arduino_Interfacing."Write to Arduino") -> ()  [unwired: 2 in, 2 out]
      }
      frame "Z STEPPER GRAB HEIGHT" {
        # ">>State Logic  >>"
        # ">>> Time cluster >>>"
        # ">>> Yaw >>>"
        # ">>> Stepper position >>>"
        # ">>> Encoders >>>"
        # ">>> Object detection >>>"
        # ">>> Ultrasonic Sensors Detect >>>"
        n174 = call "Arduino Interfacing VI.vi"("Data to Write"=I2C_MASTER_WRITE_NEW_Type_Def."zStepper 100", "AE Mode"=Arduino_Interfacing."Write to Arduino") -> ()  [unwired: 2 in, 2 out]
      }
      frame "Z STEPPER BOX HEIGHT" {
        # ">>> IR Sensors >>>"
        # ">>> Time cluster >>>"
        # ">>> Yaw >>>"
        # ">>> Stepper position >>>"
        # ">>> Encoders >>>"
        # ">>> Object detection >>>"
        # ">>> Ultrasonic Sensors Detect >>>"
        n175 = call "Arduino Interfacing VI.vi"("Data to Write"=I2C_MASTER_WRITE_NEW_Type_Def."zStepper 5k", "AE Mode"=Arduino_Interfacing."Write to Arduino") -> ()  [unwired: 2 in, 2 out]
      }
      frame "Y STEPPER CONTROL" {
        # ">>State Logic  >>"
        # ">>> yStepper command>>>"
        # ">>> Time cluster >>>"
        # ">>> Yaw >>>"
        # ">>> Stepper position >>>"
        # ">>> Encoders >>>"
        # ">>> Object detection >>>"
        # ">>> Ultrasonic Sensors Detect >>>"
        n176 = Unbundle By Name(w3694) -> ("yStepper desired"=w3693:u8)
        n177 = call "Arduino Interfacing VI.vi"("y Stepper value"=w3693, "Data to Write"=I2C_MASTER_WRITE_NEW_Type_Def."yStepper control", "AE Mode"=Arduino_Interfacing."Write to Arduino") -> ()  [unwired: 1 in, 2 out]
      }
      frame "READ STEPPER VALUES" {
        # ">>State Logic  >>"
        # ">>> Time cluster >>>"
        # ">>> Yaw >>>"
        # ">>> Stepper position >>>"
        # ">>> Encoders >>>"
        # ">>> Object detection >>>"
        # ">>> Ultrasonic Sensors Detect >>>"
        n178 = call "Arduino Interfacing VI.vi"("AE Mode"=Arduino_Interfacing."Read From Arduino") -> ("Arduino Data"=w3712:T17)  [unwired: 3 in, 1 out]
        n179 = Unbundle By Name(w3712) -> ("y Stepper Position"=w3711:u8, "z Stepper Position"=w3710:u8)
        n180 = Bundle By Name(cluster=w3715, "y Stepper Position"=w3711, "z Stepper Position"=w3710) -> (w3714:T7)
      }
      frame " -----TIMING-----" {
        # ">>State Logic  >>"
        # ">>> Time cluster >>>"
        # ">>> Yaw >>>"
        # ">>> Stepper position >>>"
        # ">>> Encoders >>>"
        # ">>> Object detection >>>"
        # ">>> Ultrasonic Sensors Detect >>>"
      }
      frame "SET TIMER 1" {
        w3731 = 1.0 ("Time Setting")
        # ">>State Logic  >>"
        # ">>> Time cluster >>>"
        # ">>> Yaw >>>"
        # ">>> Stepper position >>>"
        # ">>> Encoders >>>"
        # ">>> Object detection >>>"
        # ">>> Ultrasonic Sensors Detect >>>"
        n181 = Wait (ms)(milliseconds to wait=u32 250) -> ()  [unwired: 1 out]
        n182 = call "Elasped Timer.vi"("Time Setting"=w3731, "Action"=Elapsed_timer_control."Initialize") -> ()  [unwired: 6 in, 4 out]
        n183 = Bundle By Name(cluster=w3740, "Time up flag"=FALSE, "SET TIME TO CHECK"=w3731) -> (w3738:T3)
      }
      frame "SET TIMER 2" {
        w3747 = 2.0 ("Time Setting")
        # ">>State Logic  >>"
        # ">>> Time cluster >>>"
        # ">>> Yaw >>>"
        # ">>> Stepper position >>>"
        # ">>> Encoders >>>"
        # ">>> Object detection >>>"
        # ">>> Ultrasonic Sensors Detect >>>"
        n184 = Wait (ms)(milliseconds to wait=u32 250) -> ()  [unwired: 1 out]
        n185 = call "Elasped Timer.vi"("Time Setting"=w3747, "Action"=Elapsed_timer_control."Initialize") -> ()  [unwired: 6 in, 4 out]
        n186 = Bundle By Name(cluster=w3756, "Time up flag"=FALSE, "SET TIME TO CHECK"=w3747) -> (w3754:T3)
      }
      frame "SET TIMER 3" {
        w3763 = 3.0 ("Time Setting")
        # ">>State Logic  >>"
        # ">>> Time cluster >>>"
        # ">>> Yaw >>>"
        # ">>> Stepper position >>>"
        # ">>> Encoders >>>"
        # ">>> Object detection >>>"
        # ">>> Ultrasonic Sensors Detect >>>"
        n187 = Wait (ms)(milliseconds to wait=u32 250) -> ()  [unwired: 1 out]
        n188 = call "Elasped Timer.vi"("Time Setting"=w3763, "Action"=Elapsed_timer_control."Initialize") -> ()  [unwired: 6 in, 4 out]
        n189 = Bundle By Name(cluster=w3772, "Time up flag"=FALSE, "SET TIME TO CHECK"=w3763) -> (w3770:T3)
      }
      frame "SET TIMER 4" {
        w3779 = 4.0 ("Time Setting")
        # ">>State Logic  >>"
        # ">>> Time cluster >>>"
        # ">>> Yaw >>>"
        # ">>> Stepper position >>>"
        # ">>> Encoders >>>"
        # ">>> Object detection >>>"
        # ">>> Ultrasonic Sensors Detect >>>"
        n190 = call "Elasped Timer.vi"("Time Setting"=w3779, "Action"=Elapsed_timer_control."Initialize") -> ()  [unwired: 6 in, 4 out]
        n191 = Wait (ms)(milliseconds to wait=u32 250) -> ()  [unwired: 1 out]
        n192 = Bundle By Name(cluster=w3788, "Time up flag"=FALSE, "SET TIME TO CHECK"=w3779) -> (w3786:T3)
      }
      frame "SET TIMER 5" {
        w3796 = 5.0 ("Time Setting")
        # ">>State Logic  >>"
        # ">>> Time cluster >>>"
        # ">>> Yaw >>>"
        # ">>> Stepper position >>>"
        # ">>> Encoders >>>"
        # ">>> Object detection >>>"
        # ">>> Ultrasonic Sensors Detect >>>"
        n193 = call "Elasped Timer.vi"("Time Setting"=w3796, "Action"=Elapsed_timer_control."Initialize") -> ("Time Out?!"=w3795:bool)  [unwired: 6 in, 3 out]
        n194 = Wait (ms)(milliseconds to wait=u32 250) -> ()  [unwired: 1 out]
        n195 = Bundle By Name(cluster=w3804, "Time up flag"=w3795, "SET TIME TO CHECK"=w3796) -> (w3803:T3)
      }
      frame "START TIMER" {
        # ">>State Logic  >>"
        # ">>> Time cluster >>>"
        # ">>> Yaw >>>"
        # ">>> Stepper position >>>"
        # ">>> Encoders >>>"
        # ">>> Object detection >>>"
        # ">>> Ultrasonic Sensors Detect >>>"
        n196 = call "Elasped Timer.vi"("Action"=Elapsed_timer_control."Start") -> ("Time Out?!"=w3815:bool)  [unwired: 7 in, 3 out]
        n197 = Bundle By Name(cluster=w3818, "Time up flag"=w3815) -> (w3817:T3)
      }
      frame "-----MISC-----" {
        # ">>> Box Colour Detection >>>"
        # ">>> Line Sensor Cluster>>>"
        # ">>> IR Sensors >>>"
        # ">>> Time cluster >>>"
        # ">>> Object detection >>>"
        # ">>> Yaw >>>"
        # ">>> Ultrasonic Sensors Detect >>>"
        # ">>> Encoders >>>"
        # ">>> Stepper position >>>"
      }
      frame "Task 9" {
        # ">>> Box Colour Detection >>>"
        # ">>> Line Sensor Cluster>>>"
        # ">>> IR Sensors >>>"
        # ">>> Time cluster >>>"
        # ">>> Object detection >>>"
        # ">>> Yaw >>>"
        # ">>> Ultrasonic Sensors Detect >>>"
        # ">>> Encoders >>>"
        # ">>> Stepper position >>>"
        n198 = call "Colour Processing Test Env.vi"() -> ("Colour scan time out?"=w3844:bool, "Colour output boolean cluster"=w3842:T47)  [unwired: 10 in]
        n199 = Unbundle By Name(w3842) -> ("Red"=w3836:bool, "Black"=w3837:bool, "Blue"=w3838:bool, "Yellow"=w3839:bool, "Green"=w3840:bool, "No recognizable coolour"=w3841:bool)
        n200 = Bundle By Name(cluster=w3846, "Red"=w3836, "Black"=w3837, "Blue"=w3838, "Yellow"=w3839, "Green"=w3840, "Unknown"=w3841, "Image processing done"=w3844) -> (w3845:T1)
      }
    }
    "State Logic" <- w254
    "Image Processing Error" <- w221
    n201 = local read "TASK ENABLE"() -> (w248:bool)
    n202 = Not(x=w248) -> (.not. x?=w247:bool)
    n203 = case shown="True" w255 {
      tunnel: w212 -> [w286 w338]
      tunnel: w262 -> [w282 w340]
      tunnel: [w286 w338] -> w267
      tunnel: [w282 w341] -> w266
      tunnel: w263 -> [_ w336]
      tunnel: w265 -> [_ w337]
      tunnel: w260 -> [w285 w343]
      tunnel: [w285 w343] -> w259
      tunnel: "STOP TASK" -> [_ w326]
      tunnel: w254 -> [w284 w342]
      tunnel: [w284 w339] -> w253
      tunnel: w250 -> [w283 w332]
      tunnel: [w283 w332] -> w249
      tunnel: w247 -> [_ w327]
      tunnel: [w281 w324] -> w246
      tunnel: w245 -> [w281 w323]
      tunnel: w243 -> [w280 w320]
      tunnel: [w280 w320] -> w242
      tunnel: w240 -> [w279 w316]
      tunnel: [w279 w316] -> w239
      tunnel: w237 -> [w278 w314]
      tunnel: [w278 w314] -> w236
      tunnel: w234 -> [w277 w312]
      tunnel: [w277 w312] -> w233
      tunnel: w232 -> [w276 w311]
      tunnel: [w276 w310] -> w231
      tunnel: [_ w308] -> w230
      tunnel: w228 -> [w275 w306]
      tunnel: [w275 w306] -> w227
      tunnel: w226 -> [w274 w305]
      tunnel: [w274 w304] -> w225
      tunnel: w223 -> [w273 w301]
      tunnel: [w273 w301] -> w222
      tunnel: [w272 w300] -> w220
      tunnel: w218 -> [w272 w299]
      tunnel: [_ w297] -> w217
      tunnel: [_ w296] -> w216
      tunnel: [_ w295] -> w215
      tunnel: w213 -> [w271 w294]
      tunnel: [w271 w294] -> w211
      frame False {
        # ">>> Box Colour Detection >>>"
        # ">>> Line Sensor Cluster>>>"
        # ">> Item Selection Bias >>"
        # ">>State Logic Queue Reference >>"
        # ">>Action states Queue Reference >>"
        # ">>True Stop Next State >>"
        # ">>State Logic  >>"
        # ">>> IR Sensors >>>"
        # ">>> Line Sensor Cluster>>>"
        # ">>> Line Sensor Cluster>>>"
        # ">>> Motor control cluster >>>"
        # ">>> yStepper command>>>"
        # ">>> Motor control cluster >>>"
        # ">>> yStepper command>>>"
        # ">>> Motor control cluster >>>"
        # ">>> IR Sensors >>>"
        # ">>> IR Sensors >>>"
        # ">>> yStepper command>>>"
        # ">>> Time cluster >>>"
        # ">>> Yaw >>>"
        # ">>> Stepper position >>>"
        # ">>> Encoders >>>"
        # ">>> Object detection >>>"
        # ">>> Ultrasonic Sensors Detect >>>"
        # ">>> Time cluster >>>"
        # ">>> Yaw >>>"
        # ">>> Stepper position >>>"
        # ">>> Encoders >>>"
        # ">>> Object detection >>>"
        # ">>> Ultrasonic Sensors Detect >>>"
      }
      frame True {
        # ">>State Logic Queue Reference >>"
        # ">>> Box Colour Detection >>>"
        # ">> Item Selection Bias >>"
        # ">>> IR Sensors >>>"
        # ">>> Line Sensor Cluster>>>"
        # ">>> Line Sensor Cluster>>>"
        # ">>> Motor control cluster >>>"
        # ">>> yStepper command>>>"
        # ">>> IR Sensors >>>"
        # ">>> Motor control cluster >>>"
        # ">>State Logic Queue Reference >>"
        # ">>Timeout>>"
        # ">>> yStepper command>>>"
        # ">>> Time cluster >>>"
        # ">>> Object detection >>>"
        # ">>> Yaw >>>"
        # ">>> Ultrasonic Sensors Detect >>>"
        # ">>> Encoders >>>"
        # ">>> Stepper position >>>"
        # ">>State Logic  >>"
        # ">>True Stop Next State >>"
        # ">>Action Queue>>"
        # ">> Manual override >>"
        # ">>> Time cluster >>>"
        # ">>> Yaw >>>"
        # ">>> Stepper position >>>"
        # ">>> Encoders >>>"
        # ">>> Object detection >>>"
        # ">>> Ultrasonic Sensors Detect >>>"
        # ">>Action Queue>>"
        # ">>State Logic Queue Reference >>"
        n204 = Or(x=w326, y=w327) -> (x .or. y?=w325:bool)
        n205 = Unbundle By Name(w306) -> ("Left IR Sensor"=w307:dbl, "Arm IR Sensor"=w303:dbl, "Bottom IR Sensor"=w298:dbl)
        n206 = Unbundle By Name(w301) -> ("Line Detected?"=w302:bool)
        n207 = Unbundle By Name(w312) -> ("Time up flag"=w313:bool)
        n208 = Unbundle By Name(w314) -> ("Yaw"=w315:dbl, "Compass"=w309:dbl)
        n209 = Unbundle By Name(w316) -> ("y Stepper Position"=w318:u8, "z Stepper Position"=w317:u8)
        n210 = Unbundle By Name(w332) -> ("xDistance"=w329:dbl, "yDistance"=w330:dbl, "wDistance"=w331:dbl)
        n211 = Unbundle By Name(w320) -> ("Recognized Object"=w319:bool, "Object X coordinate"=w322:dbl, "Object Y coordinate"=w321:dbl)
        n212 = Unbundle By Name(w343) -> ("PING_A"=w335:u8, "PING_B"=w334:u8, "PING_C"=w333:u8, "PING_D"=w328:u8)
        n213 = Unbundle By Name(w294) -> ("Red"=w293:bool, "Black"=w292:bool, "Blue"=w291:bool, "Yellow"=w290:bool, "Green"=w289:bool, "Unknown"=w288:bool, "Image processing done"=w287:bool)
        n214 = case shown="38" w342 {
          tunnel: [w348 w360 w374 w385 w503 w520 w566 w603 w658 w700 w748 w792 w847 w895 w939 w999 w1040 w1083 w1132 w1175 w1228 w1266 w1318 w1362 w1406 w1436 w1454 w1500 w1541 w1590 w1643 w1682 w1731 w1774 w1827 w1865 w1917 w1953 w2002 w2045 w2095 w2139 w2182 w2237 w2274 w2322 w2361 w2403 w2458 w2512 w2550 w2596 w2645 w2686 w2730 w2778 w2824 w2871 w2912] -> w341
          tunnel: w340 -> [w348 w363 w375 w388 w505 w521 w567 w612 w656 w704 w749 w798 w840 w898 w946 w989 w1043 w1089 w1131 w1178 w1218 w1272 w1308 w1357 w1397 w1436 w1444 w1503 w1547 w1589 w1642 w1688 w1730 w1777 w1817 w1871 w1907 w1957 w2009 w2050 w2100 w2144 w2184 w2235 w2275 w2323 w2363 w2413 w2468 w2511 w2554 w2602 w2644 w2690 w2734 w2782 w2831 w2876 w2922]
          tunnel: [State_Type_Definitions,_for_0.26g_versions_and_later_2."Idle" ("Enum") State_Type_Definitions,_for_0.26g_versions_and_later_2."Idle" ("Enum") w370 w387 State_Type_Definitions,_for_0.26g_versions_and_later_2."Shutdown" ("Enum") w522 w568 w610 w659 w701 w747 w793 w846 w896 w941 w998 w1041 w1090 w1133 w1177 w1227 w1273 w1317 w1363 w1398 State_Type_Definitions,_for_0.26g_versions_and_later_2."Idle" ("Enum") w1453 w1501 w1548 w1591 w1644 w1689 w1732 w1776 w1826 w1872 w1916 w1954 w2003 w2046 w2096 w2140 w2181 w2238 w2273 w2321 w2362 w2408 w2469 w2513 w2551 w2597 w2646 w2687 w2731 w2779 w2825 w2872 w2917] -> w339
          tunnel: w338 -> [_ _ w373 w391 _ w526 w573 w606 w655 w705 w756 w797 w844 w899 w945 w996 w1038 w1088 w1129 w1179 w1225 w1271 w1315 w1360 w1405 _ w1451 w1498 w1546 w1587 w1640 w1687 w1728 w1778 w1824 w1870 w1914 w1961 w2008 w2053 w2103 w2147 w2192 w2234 w2276 w2316 w2364 w2412 w2467 w2510 w2558 w2601 w2643 w2694 w2735 w2785 w2830 w2879 w2921]
          tunnel: w337 -> [_ _ _ w390 _ w525 w572 w605 w654 w706 w755 w796 w843 w892 w944 w995 w1037 w1087 w1128 w1180 w1224 w1270 w1314 w1359 w1403 _ w1450 w1497 w1545 w1586 w1639 w1686 w1727 w1779 w1823 w1869 w1913 w1956 w2007 w2052 w2102 w2146 w2190 w2233 w2277 w2317 w2365 w2411 w2466 w2509 w2557 w2600 w2642 w2693 w2736 w2781 w2829 w2878 w2920]
          tunnel: w336 -> [_ _ w372 w386 _ w524 w571 w604 w653 w707 w754 w795 w842 w891 w943 w997 w1039 w1086 w1127 w1181 w1226 w1269 w1316 w1358 w1404 _ w1452 w1499 w1544 w1585 w1638 w1685 w1726 w1780 w1825 w1868 w1915 w1960 w2006 w2051 w2101 w2145 w2191 w2232 w2278 w2318 w2366 w2410 w2465 w2508 w2556 w2599 w2641 w2692 w2737 w2784 w2828 w2877 w2919]
          tunnel: w325 -> [_ _ _ _ _ w511 w565 w611 w652 w708 w751 w791 w845 w897 w947 w990 w1044 w1084 w1130 w1182 w1219 w1267 w1309 w1361 w1401 _ w1445 w1504 w1542 w1588 w1641 w1683 w1729 w1781 w1818 w1866 w1908 w1959 w2001 w2049 w2099 w2143 w2186 w2231 w2279 w2319 w2367 w2409 w2464 w2507 w2555 w2598 w2640 w2691 w2738 w2783 w2823 w2875 w2918]
          tunnel: w335 -> [_ _ _ _ _ _ _ _ _ _ _ _ _ _ _ _ _ _ _ _ _ _ _ _ _ _ _ _ _ _ _ _ _ _ _ _ _ _ _ _ _ _ _ _ _ _ _ _ _ _ _ _ _ _ _ _ _ _ _]
          tunnel: w334 -> [_ _ _ _ _ _ _ _ w651 _ _ _ w836 w880 w937 _ _ _ _ _ _ _ _ _ _ _ _ w1490 _ _ _ _ _ _ _ _ _ _ _ _ _ _ _ _ _ _ _ _ w2462 _ _ _ _ _ _ _ _ _ _]
          tunnel: w333 -> [_ _ _ _ _ _ _ _ w650 _ _ _ w837 w881 w938 _ _ _ _ _ _ _ _ _ _ _ _ w1491 _ _ _ _ _ _ _ _ _ _ _ _ _ _ _ _ _ _ _ _ w2463 _ _ _ _ _ _ _ _ _ _]
          tunnel: w331 -> [_ _ _ _ _ _ _ _ _ _ w753 _ _ _ _ _ _ _ _ _ _ _ _ _ _ _ _ _ _ _ _ _ _ _ _ _ _ _ _ _ _ _ _ _ _ _ _ w2406 _ _ _ _ _ _ _ _ _ _ w2915]
          tunnel: w330 -> [_ _ _ _ _ w519 w564 _ _ w699 _ _ _ _ w942 _ _ _ _ _ _ _ _ _ _ _ _ _ _ _ _ _ _ _ _ _ _ _ _ _ _ _ _ _ _ _ _ _ w2454 _ _ _ _ _ _ _ _ _ _]
          tunnel: w329 -> [_ _ _ _ _ _ _ _ _ _ _ _ _ w886 _ _ _ _ _ _ _ _ _ _ _ _ _ _ _ _ w1629 _ _ _ _ _ _ _ _ _ _ _ _ w2224 _ _ _ _ _ _ _ _ w2639 _ _ _ _ _ _]
          tunnel: w328 -> [_ _ _ _ _ _ _ _ _ _ _ _ _ _ _ _ _ _ _ _ _ _ _ _ _ _ _ _ _ _ _ _ _ _ _ _ _ _ _ _ _ _ _ _ _ _ _ _ _ _ _ _ _ _ _ _ _ _ _]
          tunnel: [State_Type_Definitions,_for_0.26g_versions_and_later_2."Idle" ("Enum") State_Type_Definitions,_for_0.26g_versions_and_later_2."Idle" ("Enum") State_Type_Definitions,_for_0.26g_versions_and_later_2."Idle" ("Enum") State_Type_Definitions,_for_0.26g_versions_and_later_2."Idle" ("Enum") State_Type_Definitions,_for_0.26g_versions_and_later_2."Shutdown" ("Enum") w517 w562 w609 w657 w702 w744 w790 w839 w894 w940 w1000 w1042 w1082 w1134 w1176 w1229 w1265 w1319 w1364 w1399 w1438 w1455 w1502 w1540 w1592 w1645 w1681 w1733 w1775 w1828 w1864 w1918 w1955 w2004 w2048 w2098 w2142 w2180 w2236 w2272 w2320 w2360 w2407 w2470 w2514 w2552 w2595 w2647 w2688 w2732 w2780 w2826 w2874 w2916] -> w324
          tunnel: w323 -> [_ _ w370 _ _ _ _ _ _ _ _ _ _ _ _ _ _ _ _ _ _ _ _ _ _ w1438 _ _ _ _ _ _ _ _ _ _ _ _ _ _ _ _ _ _ _ _ _ _ _ _ _ _ _ _ _ _ _ _ _]
          tunnel: w319 -> [_ _ _ _ _ _ _ _ _ _ _ _ _ _ _ _ _ _ _ _ _ _ _ _ w1400 _ _ _ _ _ _ _ _ _ _ _ _ _ _ _ _ _ _ _ _ _ _ _ _ _ _ _ _ _ _ _ _ _ _]
          tunnel: w322 -> [_ _ _ _ _ _ _ _ _ _ _ _ _ _ _ _ _ _ _ _ _ _ _ _ _ _ _ _ _ _ w1635 _ _ _ _ _ _ _ _ _ _ _ _ _ _ _ _ _ _ _ _ _ _ _ _ _ _ _ _]
          tunnel: w321 -> [_ _ _ _ _ _ _ _ _ _ _ _ _ _ _ _ _ _ _ w1171 _ _ _ _ _ _ _ _ _ _ _ _ _ w1770 _ _ _ _ _ _ _ _ _ _ _ _ _ _ _ _ _ _ _ _ _ _ _ _ _]
          tunnel: w318 -> [_ _ _ _ _ _ _ _ _ _ _ _ _ _ _ _ _ _ _ w1170 _ _ _ _ _ _ _ _ _ _ _ _ _ w1769 _ _ _ _ _ _ _ _ _ _ _ _ _ _ _ _ _ _ _ _ _ _ _ _ _]
          tunnel: w317 -> [_ _ _ _ _ _ _ w608 _ _ _ w788 _ _ _ w993 _ w1078 _ _ w1222 _ w1312 w1356 _ _ w1448 _ _ _ _ _ _ _ w1821 _ w1911 w1958 _ _ _ _ _ _ _ _ _ _ _ _ _ _ _ _ _ _ _ _ _]
          tunnel: w315 -> [_ _ _ _ _ _ _ _ _ _ _ _ _ _ _ _ _ _ _ _ _ _ _ _ _ _ _ _ _ _ _ _ _ _ _ _ _ _ _ _ _ _ _ _ _ _ _ _ _ _ _ _ _ _ _ _ _ _ _]
          tunnel: w313 -> [_ _ _ _ _ _ _ _ _ _ _ _ _ _ _ _ w1032 _ w1124 _ _ w1263 _ _ _ _ _ _ w1538 w1582 _ w1679 w1723 _ _ w1862 _ _ _ _ _ _ _ _ _ w2315 w2359 _ _ _ w2553 w2594 _ w2689 w2733 _ _ _ _]
          tunnel: w311 -> [w346 w358 w369 w383 w501 w516 w561 w607 w649 w703 w743 w789 w838 w890 w936 w988 w1035 w1081 w1125 w1173 w1217 w1264 w1307 w1353 w1396 w1439 w1443 w1495 w1539 w1583 w1636 w1680 w1724 w1772 w1816 w1863 w1906 w1952 w2005 w2047 w2097 w2141 w2189 w2230 w2281 w2325 w2369 w2415 w2472 w2516 w2560 w2604 w2652 w2696 w2740 w2777 w2827 w2873 w2924]
          tunnel: [w346 w357 w369 w383 w501 w516 w561 w607 w649 w703 w743 w789 w838 w890 w936 w988 w1035 w1081 w1125 w1172 w1217 w1264 w1307 w1353 w1396 w1439 w1443 w1495 w1539 w1583 w1636 w1680 w1724 w1771 w1816 w1863 w1906 w1952 w2005 w2047 w2097 w2141 w2189 w2230 w2281 w2325 w2369 w2415 w2472 w2516 w2560 w2604 w2652 w2696 w2740 w2777 w2827 w2873 w2924] -> w310
          tunnel: w309 -> [_ _ _ _ _ _ _ _ _ _ _ _ _ _ _ _ _ _ _ _ _ _ _ _ _ _ _ _ _ _ _ _ _ _ _ _ _ _ w2000 _ _ _ _ _ _ _ _ _ _ _ _ _ _ _ _ _ w2822 _ _]
          tunnel: [_ _ _ TRUE _ _ _ _ _ _ _ _ _ _ _ _ _ _ _ _ _ _ _ _ _ _ _ _ _ _ _ _ _ _ _ _ _ _ _ _ _ _ _ _ _ _ _ _ _ _ _ _ _ _ _ _ _ _ _] -> w308
          tunnel: w307 -> [_ _ _ _ _ _ _ _ _ _ _ _ _ _ _ _ _ _ _ _ _ _ _ _ _ _ _ _ _ _ _ _ _ _ _ _ _ _ _ _ _ _ _ _ _ _ _ _ _ _ _ _ _ _ _ _ _ _ _]
          tunnel: w305 -> [w345 w355 w368 w381 w500 w515 w560 w602 w648 w696 w742 w785 w831 w879 w935 w987 w1034 w1080 w1123 w1167 w1216 w1262 w1306 w1352 w1395 w1440 w1442 w1488 w1537 w1581 w1632 w1678 w1722 w1766 w1815 w1861 w1905 w1951 w1996 w2044 w2094 w2138 w2188 w2229 w2283 w2327 w2371 w2417 w2474 w2518 w2562 w2606 w2654 w2698 w2742 w2776 w2818 w2870 w2926]
          tunnel: [w345 w354 w368 w381 w500 w515 w560 w602 w648 w696 w742 w785 w831 w879 w935 w987 w1034 w1080 w1123 w1167 w1216 w1262 w1306 w1352 w1395 w1440 w1442 w1488 w1537 w1581 w1631 w1678 w1722 w1766 w1815 w1861 w1905 w1951 w1996 w2044 w2094 w2138 w2188 w2229 w2283 w2327 w2371 w2417 w2474 w2518 w2562 w2606 w2654 w2698 w2742 w2776 w2818 w2870 w2926] -> w304
          tunnel: w303 -> [_ _ _ _ _ _ _ _ _ _ _ _ _ _ _ _ _ _ _ _ _ _ _ _ _ _ _ _ _ _ _ _ _ _ _ _ _ _ _ _ w2092 _ _ _ _ _ _ _ w2460 _ _ _ _ _ _ _ _ _ _]
          tunnel: w302 -> [_ _ _ _ _ w512 _ _ _ _ _ _ _ _ w933 _ _ _ _ _ _ _ _ _ _ _ _ _ _ _ _ _ _ _ _ _ _ _ _ w2043 _ w2136 _ w2225 _ _ _ _ _ w2506 _ _ w2638 _ _ _ _ _ _]
          tunnel: [w344 w350 w367 w380 w499 w514 w559 w601 w647 w695 w741 w784 w830 w878 w934 w986 w1033 w1079 w1122 w1166 w1215 w1261 w1305 w1351 w1394 w1435 w1441 w1487 w1536 w1580 w1624 w1677 w1721 w1765 w1814 w1860 w1904 w1950 w1995 w2042 w2091 w2137 w2187 w2228 w2282 w2326 w2370 w2416 w2473 w2517 w2561 w2605 w2653 w2697 w2741 w2775 w2817 w2869 w2925] -> w300
          tunnel: w299 -> [w344 w350 w367 _ w499 w514 w559 w601 w647 w695 w741 w784 w830 w878 w934 w986 w1033 w1079 w1122 w1166 w1215 w1261 w1305 w1351 w1394 w1435 w1441 w1487 w1536 w1580 w1624 w1677 w1721 w1765 w1814 w1860 w1904 w1950 w1995 w2042 w2091 w2137 w2187 w2228 w2282 w2326 w2370 w2416 w2473 w2517 w2561 w2605 w2653 w2697 w2741 w2775 w2817 w2869 w2925]
          tunnel: w298 -> [_ _ _ _ _ _ _ _ _ _ _ _ _ _ _ _ _ _ _ _ _ _ _ _ _ _ _ _ _ _ _ _ _ _ _ _ _ _ _ _ w2090 _ _ _ _ _ _ _ _ _ _ _ _ _ _ _ _ w2866 _]
          tunnel: [_ _ _ _ _ _ _ _ w646 _ _ _ _ _ _ _ _ _ _ _ _ _ _ _ _ _ _ _ _ _ _ _ _ _ _ _ _ _ _ _ _ _ _ _ _ _ _ _ w2449 _ _ _ _ _ _ _ _ _ _] -> w297
          tunnel: [_ _ _ _ _ _ _ _ _ _ _ _ _ _ _ _ _ _ _ _ _ _ _ _ _ _ _ _ _ _ _ _ _ _ _ _ _ _ _ _ w2088 _ _ _ _ _ _ _ _ _ _ _ _ _ _ _ _ w2864 _] -> w296
          tunnel: [_ _ _ _ _ _ _ _ _ _ _ _ _ _ _ _ _ _ _ _ _ _ _ _ _ _ _ _ _ _ _ _ _ _ _ _ _ _ _ _ w2087 _ _ _ _ _ _ _ _ _ _ _ _ _ _ _ _ _ _] -> w295
          tunnel: w293 -> [_ _ _ _ _ _ _ _ _ _ _ _ _ _ _ _ _ _ _ _ _ _ _ _ _ _ _ _ _ _ _ _ _ _ _ _ _ _ _ _ _ _ _ _ _ _ _ _ _ _ _ _ _ _ _ _ _ _ _]
          tunnel: w292 -> [_ _ _ _ _ _ _ _ _ _ _ _ _ _ _ _ _ _ _ _ _ _ _ _ _ _ _ _ _ _ _ _ _ _ _ _ _ _ _ _ _ _ _ _ _ _ _ _ _ _ _ _ _ _ _ _ _ _ _]
          tunnel: w291 -> [_ _ _ _ _ _ _ _ _ _ _ _ _ _ _ _ _ _ _ _ _ _ _ _ _ _ _ _ _ _ _ _ _ _ _ _ _ _ _ _ _ _ _ _ _ _ _ _ _ _ _ _ _ _ _ _ _ _ _]
          tunnel: w290 -> [_ _ _ _ _ _ _ _ _ _ _ _ _ _ _ _ _ _ _ _ _ _ _ _ _ _ _ _ _ _ _ _ _ _ _ _ _ _ _ _ _ _ _ _ _ _ _ _ _ _ _ _ _ _ _ _ _ _ _]